vi "run_pharmaBotExp_v0.015.vi"(0 "data in":T12={"daq_ao 1"="Dev1/ao0", "daq_ai 1"="Dev1/ai0", "experiment day folder"=path "C:/multiBot/data/debug/testing", "Multiclamp init error"=0, "Multiclamp Handle Out"=10225184, "sampling rate (Hz)"=20000, "trial name"="t1"}, 1 "auto run?":bool=TRUE, 3 "which manipulator":T13(ring), 4 "HEK/slice options":enum16{"slice", "HEK"}(ring), 5 "error in":errorcluster, 6 "Validate after Experiment":bool, 7 "common cluster":T9, 11 "individual controls in":T8, 13 "images":T3={"slice image"="remote image 000000001461186C", "pipette template"="remote image 000000001461152C", "found pipette"=refnum, "pipette mask for cell tracker"=refnum, "cell images ref"=refnum}) -> (10 "Cell Looks Good?":bool=TRUE, 12 "ValidationOutputCluster":T5(array[cluster]), 14 "ValidationResults":waveform(dbl)[][](array[waveform]), 15 "ValidationPos1":T6(array[ring]), 16 "Exp. Terminated":bool, 17 "ValidationPos2":T6(array[ring]), 18 "ValidationWaveform":waveform(dbl)[](array[waveform]), 19 "error out":errorcluster)   [LabVIEW 2015] (continued)
  T24 = cluster{"Which Position to use for Experiment":enum16{"Jumper Safe Position", "Experiment Safe Position", "Jumper Position A", "Jumper Position B", "Jumper Position C", "Jumper Position o-A", "Jumper Position A-o", "Jumper Position A-B", "Jumper Position B-A", "Jumper Position B-C", "Jumper Position C-B", "Jumper Position C-o", "Jumper Position o-C", "Don't Move"}, "Duration (s)":dbl, "Delay (s)":dbl, "Ramp Slope (mV/s)":dbl, "Voltage Start (mV)":dbl, "Replicates":dbl, "Voltage End (mV)":dbl, "Ramp Duration (s)":dbl, "Vholding (mV)":dbl, "Valve 1 Position":i16, "Valve 2 Position":i16, "Valve 3 Position":i16, "valve 1 used now?":bool, "valve 2 used now?":bool, "valve 3 used now? ":bool, "Maintain Final Voltage until end?":bool, "protocol Preview":waveform(dbl)[]}
  T25 = cluster{"Which Position to use for Experiment":enum16{"Jumper Safe Position", "Experiment Safe Position", "Jumper Position A", "Jumper Position B", "Jumper Position C", "Jumper Position o-A", "Jumper Position A-o", "Jumper Position A-B", "Jumper Position B-A", "Jumper Position B-C", "Jumper Position C-B", "Jumper Position C-o", "Jumper Position o-C", "Don't Move"}, "Duration (s)":dbl, "Delay (s)":dbl, "Pulse 2 (s)":dbl, "Pulse 1 (mV)":dbl, "Replicates":dbl, "Pulse 1 (s)":dbl, "Pulse 2 (mV)":dbl, "Vholding (mV)":dbl, "Valve 1 Position":i16, "Valve 2 Position":i16, "Valve 3 Position":i16, "valve 1 used now?":bool, "valve 2 used now?":bool, "valve 3 used now? ":bool, "Maintain Final Voltage until end?":bool, "delta Pulse 1 (mV)":dbl, "delta Pulse 2 (mV)":dbl, "Sweeps":dbl, "Final Pulse 1 (mV)":dbl, "Final Pulse 2 (mV)":dbl, "protocol Preview":waveform(dbl)[]}
  T26 = cluster{"Which Position to use for Experiment":enum16{"Jumper Safe Position", "Experiment Safe Position", "Jumper Position A", "Jumper Position B", "Jumper Position C", "Jumper Position o-A", "Jumper Position A-o", "Jumper Position A-B", "Jumper Position B-A", "Jumper Position B-C", "Jumper Position C-B", "Jumper Position C-o", "Jumper Position o-C", "Don't Move"}, "Start Position (N)":string, "Jump Position (m)":string, "Duration (s)":dbl, "Delay (s)":dbl, "Pulse Width (s)":dbl, "Valve 1 Position":i16, "Valve 2 Position":i16, "Replicates":dbl, "Pulse Period (s)":dbl, "Vholding (mV)":dbl, "Number of Pulses":dbl, "valve 1 used now?":bool, "valve 2 used now?":bool, "valve 3 used now? ":bool, "Valve 3 Position":i16, "protocol Preview":waveform(dbl)[]}
  T27 = cluster{"Which Position to use for Experiment":enum16{"Jumper Safe Position", "Experiment Safe Position", "Jumper Position A", "Jumper Position B", "Jumper Position C", "Jumper Position o-A", "Jumper Position A-o", "Jumper Position A-B", "Jumper Position B-A", "Jumper Position B-C", "Jumper Position C-B", "Jumper Position C-o", "Jumper Position o-C", "Don't Move"}, "Start Position (N)":string, "Jump Position (m)":string, "Duration (s)":dbl, "Delay (s)":dbl, "Pulse Width (s)":dbl, "Replicates":dbl, "Pulse Delay (s)":dbl, "Pulse Delta Delay (s)":dbl, "Vholding (mV)":dbl, "Valve 1 Position":i16, "Valve 2 Position":i16, "valve 1 used now?":bool, "valve 2 used now?":bool, "valve 3 used now? ":bool, "Valve 3 Position":i16, "protocol Preview":waveform(dbl)[]}
  T28 = cluster{"Start Position (N)":enum16{"Jumper Safe Position", "Experiment Safe Position", "Jumper Position A", "Jumper Position B", "Jumper Position C", "Jumper Position o-A", "Jumper Position A-o", "Jumper Position A-B", "Jumper Position B-A", "Jumper Position B-C", "Jumper Position C-B", "Jumper Position C-o", "Jumper Position o-C", "Don't Move"}, "Duration (s)":dbl, "Delay (s)":dbl, "Pulse Width (s)":dbl, "Valve 1 Position":i16, "Valve 2 Position":i16, "Replicates":dbl, "Jump Position (m)":enum16{"Jumper Safe Position", "Experiment Safe Position", "Jumper Position A", "Jumper Position B", "Jumper Position C", "Jumper Position o-A", "Jumper Position A-o", "Jumper Position A-B", "Jumper Position B-A", "Jumper Position B-C", "Jumper Position C-B", "Jumper Position C-o", "Jumper Position o-C", "Don't Move"}, "Vholding (mV)":dbl, "Valve 3 Position":i16, "valve 1 used now?":bool, "valve 2 used now?":bool, "valve 3 used now? ":bool, "protocol Preview":waveform(dbl)[]}
  T29 = cluster{"Which Position to use for Experiment":enum16{"Jumper Safe Position", "Experiment Safe Position", "Jumper Position A", "Jumper Position B", "Jumper Position C", "Jumper Position o-A", "Jumper Position A-o", "Jumper Position A-B", "Jumper Position B-A", "Jumper Position B-C", "Jumper Position C-B", "Jumper Position C-o", "Jumper Position o-C", "Don't Move"}, "Duration (s)":dbl, "Valve 1 Position":i16, "Valve 2 Position":i16, "Replicates":dbl, "Vholding (mV)":dbl, "Valve 3 Position":i16, "valve 1 used now?":bool, "valve 2 used now?":bool, "valve 3 used now? ":bool, "Record During Solution Change?":bool}
  T30 = cluster{"Start Position (N)":enum16{"Jumper Safe Position", "Experiment Safe Position", "Jumper Position A", "Jumper Position B", "Jumper Position C", "Jumper Position o-A", "Jumper Position A-o", "Jumper Position A-B", "Jumper Position B-A", "Jumper Position B-C", "Jumper Position C-B", "Jumper Position C-o", "Jumper Position o-C"}, "Duration (s)":dbl, "Delay (s)":dbl, "Valve 1 Position":i16, "Valve 2 Position":i16, "Replicates":dbl, "Vholding (mV)":dbl, "Valve 3 Position":i16, "valve 1 used now?":bool, "valve 2 used now?":bool, "valve 3 used now? ":bool, "Jump Position Array":enum16{"Jumper Safe Position", "Experiment Safe Position", "Jumper Position A", "Jumper Position B", "Jumper Position C", "Jumper Position o-A", "Jumper Position A-o", "Jumper Position A-B", "Jumper Position B-A", "Jumper Position B-C", "Jumper Position C-B", "Jumper Position C-o", "Jumper Position o-C"}[], "Position Dwell Time (s)":dbl[], "protocol Preview":waveform(dbl)[]}
  T31 = cluster{"Which Position to use for Experiment":enum16{"Jumper Safe Position", "Experiment Safe Position", "Jumper Position A", "Jumper Position B", "Jumper Position C", "Jumper Position o-A", "Jumper Position A-o", "Jumper Position A-B", "Jumper Position B-A", "Jumper Position B-C", "Jumper Position C-B", "Jumper Position C-o", "Jumper Position o-C", "Don't Move"}, "Duration (s)":dbl, "Delay (s)":dbl, "Pulse 2 (s)":dbl, "Pulse 1 (pA)":dbl, "Replicates":dbl, "Pulse 1 (s)":dbl, "Pulse 2 (pA)":dbl, "Iholding (pA)":dbl, "Valve 1 Position":i16, "Valve 2 Position":i16, "Valve 3 Position":i16, "valve 1 used now?":bool, "valve 2 used now?":bool, "valve 3 used now? ":bool, "Maintain Final Voltage until end?":bool, "delta Pulse 1 (pA)":dbl, "delta Pulse 2 (pA)":dbl, "Sweeps":dbl, "Final Pulse 1 (pA)":dbl, "Final Pulse 2 (pA)":dbl, "protocol Preview":waveform(dbl)[]}
  T32 = cluster{"Which Position to use for Experiment":enum16{"Jumper Safe Position", "Experiment Safe Position", "Jumper Position A", "Jumper Position B", "Jumper Position C", "Jumper Position o-A", "Jumper Position A-o", "Jumper Position A-B", "Jumper Position B-A", "Jumper Position B-C", "Jumper Position C-B", "Jumper Position C-o", "Jumper Position o-C", "Don't Move"}, "Duration (s)":dbl, "Delay (s)":dbl, "Ramp Slope (pA/s)":dbl, "Current Start (pA)":dbl, "Replicates":dbl, "Current End (pA)":dbl, "Ramp Duration (s)":dbl, "Iholding (pA)":dbl, "Valve 1 Position":i16, "Valve 2 Position":i16, "Valve 3 Position":i16, "valve 1 used now?":bool, "valve 2 used now?":bool, "valve 3 used now? ":bool, "Maintain Final Voltage until end?":bool, "protocol Preview":waveform(dbl)[]}
  T33 = cluster{"Which Position to use for Experiment":enum16{"Jumper Safe Position", "Experiment Safe Position", "Jumper Position A", "Jumper Position B", "Jumper Position C", "Jumper Position o-A", "Jumper Position A-o", "Jumper Position A-B", "Jumper Position B-A", "Jumper Position B-C", "Jumper Position C-B", "Jumper Position C-o", "Jumper Position o-C", "Don't Move"}, "Duration (s)":dbl, "Valve 1 Position":i16, "Valve 2 Position":i16, "Replicates":dbl, "Iholding (pA)":dbl, "Valve 3 Position":i16, "valve 1 used now?":bool, "valve 2 used now?":bool, "valve 3 used now? ":bool, "Record During Solution Change?":bool}
  T34 = cluster{"Phase A Done":refnum<vi>, "Phase B Done":refnum<vi>, "Phase C Done":refnum<vi>, "Phase D Done":refnum<vi>, "Phase E Done":refnum<vi>, "Phase F Done":refnum<vi>, "Phase G Done":refnum<vi>, "Phase H Done":refnum<vi>, "Phase I Done":refnum<vi>, "Phase J Done":refnum<vi>, "Phase K Done":refnum<vi>, "Phase L Done":refnum<vi>}
  T35 = cluster{"time of Last V1 Change":refnum<vi>, "time of Last V2 Change":refnum<vi>, "time of Last V3 Change":refnum<vi>}
  T36 = typedef "transform_cluster_actuator.ctl" = cluster{"s":refnum<vi>, "manip 1":refnum<vi>, "manip 2":refnum<vi>, "manip 3":refnum<vi>, "manip 4":refnum<vi>}
  T37 = typedef "transform_properties_actuators.ctl" = cluster{"theta (deg)":dbl, "X sc factor (px/step)":dbl, "Y sc factor (px/step)":dbl, "zero loc (x,y,z)":dbl[], "flip y?":bool, "flip x?":bool, "gamma (deg)":dbl, "flip z?":bool, "Z sc factor (px/step)":dbl, "actuator":T38, "safe space (steps)":i32[]}
  T38 = typedef "actuator_cluster.ctl" = cluster{"Actuator COM":refnum<visa-resource-name>, "Actuator type":T39}
  T39 = typedef "actuator_type.ctl" = enum16{"Scientifica", "Sutter", "Demo", "Off"}
  T40 = typedef "RWC_Actions.ctl" = enum16{"Read", "Write", "Read and Create"}
  T41 = enum16{"open", "replace", "create", "open or create", "replace or create", "replace or create with confirmation"}
  T42 = enum16{"Jumper Safe Position", "Experiment Safe Position", "Jumper Position A", "Jumper Position B", "Jumper Position C", "Jumper Position o-A", "Jumper Position A-o", "Jumper Position A-B", "Jumper Position B-A", "Jumper Position B-C", "Jumper Position C-B", "Jumper Position C-o", "Jumper Position o-C"}
  T43 = typedef "NI_AALBase.lvlib/Filter Passband Type.ctl" = enum32{"Lowpass", "Highpass", "Bandpass", "Bandstop"}
  T44 = enum32{"Invalid", "Standard", "Closed", "Hidden", "Minimized", "Maximized"}
  T45 = typedef "pressure_box_control.ctl" = cluster{"Pressure box COM":refnum<visa-resource-name>, "pressure box type":T46, "High pos pressure (mBar)":dbl, "Low pos pressure (mBar)":dbl, "Vacuum pressure (mBar)":dbl, "calibration":enum16{"PA_vacPump", "PA_venturi", "Neuromatics", "ilyaRig", "mightenRig"}}
  T46 = typedef "pressure_box_type.ctl" = enum16{"Neuromatics", "ProportionAir", "Demo box", "N-ProportionAir"}
diagram:
  w338 = FALSE ("Phase A")
  w339 = "" ("Phase A Exp Option")
  w340 = FALSE ("Phase A")
  # "ValidatePositions & Clean?"
  # "Analyze\nInitial\nData"
  # "SaveConfig"
  # "EndingSet"
  # "RunExperiment"
  # "StartingSet"
  # "Run QC"
  # "Move To Experiment \n          safe space"
  # "Lift Cell"
  # "RUN AUTO WC"
  # "initializing"
  # "Initalization"
  # "HEK/slice options = \"\\14\\00€\\00\\00\\00\\00\\01\\00#@\\16\\00\\02\\05slice\\03HEK\\00\\11HEK/slice options\\00\\01\\00\\00\\00\\01\\00\\00\\00\\00\"\nHEK/slice options string = \"\\14\\00€\\00\\00\\00\\00\\01\\00\"@0ÿÿÿÿ\\18HEK/slice options string\\00\\00\\01\\00\\00\\00\\00\\00\\03HEK\\00\\00\\00\\00\""
  # "PLOTS"
  # "MISC"
  # "create reference for vclamp, iclamp plots\nsave as folder"
  # "load initial values"
  # "HOLDING"
  # "repMemTest"
  n1 = control-ref of="Jump Train G"() -> (w91:refnum<vi>)
  n2 = control-ref of="Paired Pulse G"() -> (w92:refnum<vi>)
  n3 = control-ref of="Voltage Ramp G"() -> (w90:refnum<vi>)
  n4 = control-ref of="Voltage Step G"() -> (w89:refnum<vi>)
  n5 = control-ref of="Solution Change G"() -> (w88:refnum<vi>)
  n6 = control-ref of="Single Jump G"() -> (w87:refnum<vi>)
  n7 = control-ref of="Single Manip Jump G"() -> (w86:refnum<vi>)
  n8 = control-ref of="Current Pulse G"() -> (w22:refnum<vi>)
  n9 = control-ref of="Current Ramp G"() -> (w21:refnum<vi>)
  n10 = control-ref of="Gap Free Iclamp G"() -> (w20:refnum<vi>)
  n11 = control-ref of="Gap Free G"() -> (w85:refnum<vi>)
  n12 = control-ref of="Multi Manip Jump G"() -> (w84:refnum<vi>)
  n13 = control-ref of="Voltage Pulse G"() -> (w83:refnum<vi>)
  n14 = control-ref of="PhaseG Experiment Option"() -> (w352:refnum<vi>)
  n15 = control-ref of="PhaseA Experiment Option"() -> (w390:refnum<vi>)
  n16 = control-ref of="Gap Free Iclamp A"() -> (w38:refnum<vi>)
  n17 = control-ref of="Current Ramp A"() -> (w39:refnum<vi>)
  n18 = control-ref of="Current Pulse A"() -> (w40:refnum<vi>)
  n19 = control-ref of="Multi Manip Jump A"() -> (w311:refnum<vi>)
  n20 = control-ref of="Single Manip Jump A"() -> (w309:refnum<vi>)
  n21 = control-ref of="Voltage Pulse A"() -> (w312:refnum<vi>)
  n22 = control-ref of="Gap Free A"() -> (w310:refnum<vi>)
  n23 = control-ref of="Paired Pulse A"() -> (w303:refnum<vi>)
  n24 = control-ref of="Voltage Ramp A"() -> (w305:refnum<vi>)
  n25 = control-ref of="Voltage Step A"() -> (w306:refnum<vi>)
  n26 = control-ref of="Solution Change A"() -> (w307:refnum<vi>)
  n27 = control-ref of="Single Jump A"() -> (w308:refnum<vi>)
  n28 = control-ref of="Jump Train A"() -> (w304:refnum<vi>)
  n29 = control-ref of="Jump Train H"() -> (w101:refnum<vi>)
  n30 = control-ref of="Paired Pulse H"() -> (w102:refnum<vi>)
  n31 = control-ref of="Voltage Ramp H"() -> (w100:refnum<vi>)
  n32 = control-ref of="Voltage Step H"() -> (w99:refnum<vi>)
  n33 = control-ref of="Solution Change H"() -> (w98:refnum<vi>)
  n34 = control-ref of="Single Jump H"() -> (w97:refnum<vi>)
  n35 = control-ref of="Single Manip Jump H"() -> (w96:refnum<vi>)
  n36 = control-ref of="Gap Free H"() -> (w95:refnum<vi>)
  n37 = control-ref of="Multi Manip Jump H"() -> (w94:refnum<vi>)
  n38 = control-ref of="Voltage Pulse H"() -> (w93:refnum<vi>)
  n39 = control-ref of="Current Pulse H"() -> (w19:refnum<vi>)
  n40 = control-ref of="Current Ramp H"() -> (w18:refnum<vi>)
  n41 = control-ref of="Gap Free Iclamp H"() -> (w17:refnum<vi>)
  n42 = Build Array(w352, w92, w91, w90, w89, w88, w87, w86, w85, w84, w83, w22, w21, w20) -> (w346:refnum<vi>[])
  n43 = control-ref of="PhaseH Experiment Option"() -> (w351:refnum<vi>)
  n44 = control-ref of="PhaseB Experiment Option"() -> (w389:refnum<vi>)
  n45 = Build Array(w390, w303, w304, w305, w306, w307, w308, w309, w310, w311, w312, w40, w39, w38) -> (w384:refnum<vi>[])
  n46 = control-ref of="Paired Pulse B"() -> (w292:refnum<vi>)
  n47 = control-ref of="Jump Train B"() -> (w291:refnum<vi>)
  n48 = control-ref of="Voltage Ramp B"() -> (w290:refnum<vi>)
  n49 = control-ref of="Voltage Step B"() -> (w289:refnum<vi>)
  n50 = control-ref of="Solution Change B"() -> (w288:refnum<vi>)
  n51 = control-ref of="Single Jump B"() -> (w287:refnum<vi>)
  n52 = control-ref of="Single Manip Jump B"() -> (w286:refnum<vi>)
  n53 = control-ref of="Gap Free B"() -> (w285:refnum<vi>)
  n54 = control-ref of="Multi Manip Jump B"() -> (w284:refnum<vi>)
  n55 = control-ref of="Voltage Pulse B"() -> (w283:refnum<vi>)
  n56 = control-ref of="Current Pulse B"() -> (w37:refnum<vi>)
  n57 = control-ref of="Current Ramp B"() -> (w36:refnum<vi>)
  n58 = control-ref of="Gap Free Iclamp B"() -> (w35:refnum<vi>)
  n59 = control-ref of="A Solution1"() -> (w419:refnum<vi>)
  n60 = control-ref of="A Solution2"() -> (w418:refnum<vi>)
  n61 = control-ref of="A Solution3"() -> (w417:refnum<vi>)
  n62 = control-ref of="A Solution4"() -> (w416:refnum<vi>)
  n63 = control-ref of="A Solution5"() -> (w415:refnum<vi>)
  n64 = control-ref of="A Solution6"() -> (w414:refnum<vi>)
  n65 = control-ref of="A Solution7"() -> (w413:refnum<vi>)
  n66 = control-ref of="A Solution8"() -> (w412:refnum<vi>)
  n67 = control-ref of="Jump Train I"() -> (w111:refnum<vi>)
  n68 = control-ref of="Paired Pulse I"() -> (w112:refnum<vi>)
  n69 = control-ref of="Voltage Ramp I"() -> (w110:refnum<vi>)
  n70 = control-ref of="Voltage Step I"() -> (w109:refnum<vi>)
  n71 = control-ref of="Solution Change I"() -> (w108:refnum<vi>)
  n72 = control-ref of="Single Jump I"() -> (w107:refnum<vi>)
  n73 = control-ref of="Single Manip Jump I"() -> (w106:refnum<vi>)
  n74 = control-ref of="Gap Free I"() -> (w105:refnum<vi>)
  n75 = control-ref of="Multi Manip Jump I"() -> (w104:refnum<vi>)
  n76 = control-ref of="Voltage Pulse I"() -> (w103:refnum<vi>)
  n77 = control-ref of="Current Pulse I"() -> (w16:refnum<vi>)
  n78 = control-ref of="Current Ramp I"() -> (w15:refnum<vi>)
  n79 = control-ref of="Gap Free Iclamp I"() -> (w14:refnum<vi>)
  n80 = control-ref of="PhaseI Experiment Option"() -> (w350:refnum<vi>)
  n81 = Build Array(w351, w102, w101, w100, w99, w98, w97, w96, w95, w94, w93, w19, w18, w17) -> (w345:refnum<vi>[])
  n82 = control-ref of="Paired Pulse C"() -> (w272:refnum<vi>)
  n83 = control-ref of="Jump Train C"() -> (w271:refnum<vi>)
  n84 = control-ref of="Voltage Ramp C"() -> (w270:refnum<vi>)
  n85 = control-ref of="Voltage Step C"() -> (w269:refnum<vi>)
  n86 = control-ref of="Solution Change C"() -> (w268:refnum<vi>)
  n87 = control-ref of="Single Jump C"() -> (w267:refnum<vi>)
  n88 = control-ref of="Single Manip Jump C"() -> (w266:refnum<vi>)
  n89 = control-ref of="Gap Free C"() -> (w265:refnum<vi>)
  n90 = control-ref of="Multi Manip Jump C"() -> (w264:refnum<vi>)
  n91 = control-ref of="Current Pulse C"() -> (w34:refnum<vi>)
  n92 = control-ref of="Current Ramp C"() -> (w33:refnum<vi>)
  n93 = control-ref of="Gap Free Iclamp C"() -> (w32:refnum<vi>)
  n94 = control-ref of="Voltage Pulse C"() -> (w263:refnum<vi>)
  n95 = control-ref of="PhaseC Experiment Option"() -> (w388:refnum<vi>)
  n96 = Build Array(w389, w292, w291, w290, w289, w288, w287, w286, w285, w284, w283, w37, w36, w35) -> (w383:refnum<vi>[])
  n97 = Build Array(w419, w418, w417, w416, w415, w414, w413, w412) -> (w411:refnum<vi>[])
  n98 = control-ref of="Paired Pulse J"() -> (w122:refnum<vi>)
  n99 = control-ref of="Single Manip Jump J"() -> (w116:refnum<vi>)
  n100 = control-ref of="Voltage Ramp J"() -> (w120:refnum<vi>)
  n101 = control-ref of="Voltage Step J"() -> (w119:refnum<vi>)
  n102 = control-ref of="Solution Change J"() -> (w118:refnum<vi>)
  n103 = control-ref of="Single Jump J"() -> (w117:refnum<vi>)
  n104 = control-ref of="Jump Train J"() -> (w121:refnum<vi>)
  n105 = control-ref of="Gap Free J"() -> (w115:refnum<vi>)
  n106 = control-ref of="Multi Manip Jump J"() -> (w114:refnum<vi>)
  n107 = control-ref of="Voltage Pulse J"() -> (w113:refnum<vi>)
  n108 = control-ref of="Current Pulse J"() -> (w13:refnum<vi>)
  n109 = control-ref of="Current Ramp J"() -> (w12:refnum<vi>)
  n110 = control-ref of="Gap Free Iclamp J"() -> (w11:refnum<vi>)
  n111 = control-ref of="B Solution1"() -> (w409:refnum<vi>)
  n112 = control-ref of="B Solution2"() -> (w405:refnum<vi>)
  n113 = control-ref of="B Solution3"() -> (w404:refnum<vi>)
  n114 = control-ref of="B Solution4"() -> (w403:refnum<vi>)
  n115 = control-ref of="B Solution5"() -> (w402:refnum<vi>)
  n116 = control-ref of="B Solution6"() -> (w406:refnum<vi>)
  n117 = control-ref of="B Solution7"() -> (w407:refnum<vi>)
  n118 = control-ref of="B Solution8"() -> (w408:refnum<vi>)
  n119 = Build Array(w350, w112, w111, w110, w109, w108, w107, w106, w105, w104, w103, w16, w15, w14) -> (w344:refnum<vi>[])
  n120 = control-ref of="PhaseD Experiment Option"() -> (w387:refnum<vi>)
  n121 = control-ref of="PhaseJ Experiment Option"() -> (w349:refnum<vi>)
  n122 = Build Array(w388, w272, w271, w270, w269, w268, w267, w266, w265, w264, w263, w34, w33, w32) -> (w382:refnum<vi>[])
  n123 = control-ref of="Current Pulse D"() -> (w31:refnum<vi>)
  n124 = control-ref of="Current Ramp D"() -> (w30:refnum<vi>)
  n125 = control-ref of="Gap Free Iclamp D"() -> (w29:refnum<vi>)
  n126 = control-ref of="Paired Pulse D"() -> (w252:refnum<vi>)
  n127 = control-ref of="Jump Train D"() -> (w251:refnum<vi>)
  n128 = control-ref of="Voltage Ramp D"() -> (w250:refnum<vi>)
  n129 = control-ref of="Voltage Step D"() -> (w249:refnum<vi>)
  n130 = control-ref of="Solution Change D"() -> (w248:refnum<vi>)
  n131 = control-ref of="Single Jump D"() -> (w247:refnum<vi>)
  n132 = control-ref of="Single Manip Jump D"() -> (w246:refnum<vi>)
  n133 = control-ref of="Gap Free D"() -> (w245:refnum<vi>)
  n134 = control-ref of="Multi Manip Jump D"() -> (w244:refnum<vi>)
  n135 = control-ref of="Voltage Pulse D"() -> (w243:refnum<vi>)
  n136 = Build Array(w409, w405, w404, w403, w402, w406, w407, w408) -> (w401:refnum<vi>[])
  n137 = control-ref of="PhaseE Experiment Option"() -> (w386:refnum<vi>)
  n138 = Build Array(w387, w252, w251, w250, w249, w248, w247, w246, w245, w244, w243, w31, w30, w29) -> (w381:refnum<vi>[])
  n139 = Build Array(w349, w122, w121, w120, w119, w118, w117, w116, w115, w114, w113, w13, w12, w11) -> (w343:refnum<vi>[])
  n140 = control-ref of="PhaseK Experiment Option"() -> (w348:refnum<vi>)
  n141 = control-ref of="Paired Pulse K"() -> (w123:refnum<vi>)
  n142 = control-ref of="Single Manip Jump K"() -> (w129:refnum<vi>)
  n143 = control-ref of="Voltage Ramp K"() -> (w125:refnum<vi>)
  n144 = control-ref of="Voltage Step K"() -> (w126:refnum<vi>)
  n145 = control-ref of="Solution Change K"() -> (w127:refnum<vi>)
  n146 = control-ref of="Single Jump K"() -> (w128:refnum<vi>)
  n147 = control-ref of="Jump Train K"() -> (w124:refnum<vi>)
  n148 = control-ref of="Gap Free K"() -> (w130:refnum<vi>)
  n149 = control-ref of="Multi Manip Jump K"() -> (w131:refnum<vi>)
  n150 = control-ref of="Voltage Pulse K"() -> (w132:refnum<vi>)
  n151 = control-ref of="Current Pulse E"() -> (w28:refnum<vi>)
  n152 = control-ref of="Current Ramp E"() -> (w27:refnum<vi>)
  n153 = control-ref of="Gap Free Iclamp E"() -> (w26:refnum<vi>)
  n154 = control-ref of="Current Pulse K"() -> (w10:refnum<vi>)
  n155 = control-ref of="Current Ramp K"() -> (w9:refnum<vi>)
  n156 = control-ref of="Gap Free Iclamp K"() -> (w8:refnum<vi>)
  n157 = control-ref of="Jump Train E"() -> (w231:refnum<vi>)
  n158 = control-ref of="Voltage Ramp E"() -> (w230:refnum<vi>)
  n159 = control-ref of="Voltage Step E"() -> (w229:refnum<vi>)
  n160 = control-ref of="Solution Change E"() -> (w228:refnum<vi>)
  n161 = control-ref of="Single Jump E"() -> (w227:refnum<vi>)
  n162 = control-ref of="Single Manip Jump E"() -> (w226:refnum<vi>)
  n163 = control-ref of="Gap Free E"() -> (w225:refnum<vi>)
  n164 = control-ref of="Multi Manip Jump E"() -> (w224:refnum<vi>)
  n165 = control-ref of="Voltage Pulse E"() -> (w223:refnum<vi>)
  n166 = control-ref of="Paired Pulse E"() -> (w232:refnum<vi>)
  n167 = control-ref of="C Solution1"() -> (w399:refnum<vi>)
  n168 = control-ref of="C Solution2"() -> (w398:refnum<vi>)
  n169 = control-ref of="C Solution3"() -> (w397:refnum<vi>)
  n170 = control-ref of="C Solution4"() -> (w396:refnum<vi>)
  n171 = control-ref of="C Solution5"() -> (w395:refnum<vi>)
  n172 = control-ref of="C Solution6"() -> (w394:refnum<vi>)
  n173 = control-ref of="C Solution7"() -> (w393:refnum<vi>)
  n174 = control-ref of="C Solution8"() -> (w392:refnum<vi>)
  n175 = control-ref of="Command steps (mV)"() -> (w459:refnum<vi>)
  n176 = control-ref of="Command steps (pA)"() -> (w464:refnum<vi>)
  n177 = control-ref of="Recorded currents (pA)"() -> (w463:refnum<vi>)
  n178 = control-ref of="Recorded voltage (mV)"() -> (w462:refnum<vi>)
  n179 = Build Array(w399, w398, w397, w396, w395, w394, w393, w392) -> (w391:refnum<vi>[])
  n180 = Build Array(w348, w123, w124, w125, w126, w127, w128, w129, w130, w131, w132, w10, w9, w8) -> (w342:refnum<vi>[])
  n181 = control-ref of="PhaseF Experiment Option"() -> (w385:refnum<vi>)
  n182 = Build Array(w386, w232, w231, w230, w229, w228, w227, w226, w225, w224, w223, w28, w27, w26) -> (w380:refnum<vi>[])
  n183 = control-ref of="holding memtest"() -> (w467:refnum<vi>)
  n184 = control-ref of="Paired Pulse L"() -> (w142:refnum<vi>)
  n185 = control-ref of="Single Manip Jump L"() -> (w136:refnum<vi>)
  n186 = control-ref of="Current Pulse F"() -> (w25:refnum<vi>)
  n187 = control-ref of="Current Ramp F"() -> (w24:refnum<vi>)
  n188 = control-ref of="Gap Free Iclamp F"() -> (w23:refnum<vi>)
  n189 = control-ref of="Voltage Ramp L"() -> (w140:refnum<vi>)
  n190 = control-ref of="Voltage Step L"() -> (w139:refnum<vi>)
  n191 = control-ref of="Solution Change L"() -> (w138:refnum<vi>)
  n192 = control-ref of="Single Jump L"() -> (w137:refnum<vi>)
  n193 = control-ref of="Jump Train L"() -> (w141:refnum<vi>)
  n194 = control-ref of="Paired Pulse F"() -> (w152:refnum<vi>)
  n195 = control-ref of="Jump Train F"() -> (w151:refnum<vi>)
  n196 = control-ref of="Voltage Ramp F"() -> (w150:refnum<vi>)
  n197 = control-ref of="Voltage Step F"() -> (w149:refnum<vi>)
  n198 = control-ref of="Solution Change F"() -> (w148:refnum<vi>)
  n199 = control-ref of="Single Jump F"() -> (w147:refnum<vi>)
  n200 = control-ref of="Single Manip Jump F"() -> (w146:refnum<vi>)
  n201 = control-ref of="Gap Free F"() -> (w145:refnum<vi>)
  n202 = control-ref of="Multi Manip Jump F"() -> (w144:refnum<vi>)
  n203 = control-ref of="Voltage Pulse F"() -> (w143:refnum<vi>)
  n204 = control-ref of="repMemTest Iprot"() -> (w486:refnum<vi>)
  n205 = control-ref of="repMemTest Vprot"() -> (w485:refnum<vi>)
  n206 = control-ref of="repMemTest Iclamp memtest"() -> (w484:refnum<vi>)
  n207 = control-ref of="repMemTest Vclamp memtest"() -> (w483:refnum<vi>)
  n208 = control-ref of="repMemTest sets"() -> (w487:refnum<vi>)
  n209 = control-ref of="holding Iclamp memtest"() -> (w469:refnum<vi>)
  n210 = control-ref of="holding Vclamp memtest"() -> (w468:refnum<vi>)
  n211 = control-ref of="cell stats"() -> (w465:refnum<vi>)
  n212 = control-ref of="Gap Free L"() -> (w135:refnum<vi>)
  n213 = control-ref of="wait after init (s)"() -> (w488:refnum<vi>)
  n214 = control-ref of="wait after repMemTest set (s)"() -> (w489:refnum<vi>)
  n215 = control-ref of="Multi Manip Jump L"() -> (w134:refnum<vi>)
  n216 = control-ref of="Voltage Pulse L"() -> (w133:refnum<vi>)
  n217 = control-ref of="Current Pulse L"() -> (w7:refnum<vi>)
  n218 = control-ref of="Current Ramp L"() -> (w6:refnum<vi>)
  n219 = control-ref of="Gap Free Iclamp L"() -> (w5:refnum<vi>)
  n220 = control-ref of="status"() -> (w466:refnum<vi>)
  n221 = control-ref of="trial comments"() -> (w461:refnum<vi>)
  n222 = control-ref of="release notes"() -> (w460:refnum<vi>)
  n223 = control-ref of="PhaseL Experiment Option"() -> (w347:refnum<vi>)
  n224 = control-ref of="config file"() -> ()  [unwired: 1 out]
  n225 = control-ref of="Validate after Experiment"() -> (w2:refnum<vi>)
  n226 = control-ref of="twitter?"() -> (w4:refnum<vi>)
  n227 = control-ref of="Don't Lift?"() -> (w3:refnum<vi>)
  n228 = control-ref of="Lane C Controlled by which valve?"() -> (w400:refnum<vi>)
  n229 = control-ref of="Lane A Controlled by which valve?"() -> (w420:refnum<vi>)
  n230 = control-ref of="Lane B Controlled by which valve?"() -> (w410:refnum<vi>)
  n231 = control-ref of="How Many Experimental Phases?"() -> (w422:refnum<vi>)
  n232 = control-ref of="Lift Cell (T, F-Pull Patch)?"() -> (w421:refnum<vi>)
  n233 = Build Array(w385, w152, w151, w150, w149, w148, w147, w146, w145, w144, w143, w25, w24, w23) -> (w379:refnum<vi>[])
  n234 = Build Array(w347, w142, w141, w140, w139, w138, w137, w136, w135, w134, w133, w7, w6, w5) -> (w341:refnum<vi>[])
  n235 = control-ref of="Waveform Simulation sampling rate (Hz)"() -> (w79:refnum<vi>)
  n236 = control-ref of="Waveform Simulation Jump Filter (Hz)"() -> (w77:refnum<vi>)
  n237 = flat-sequence {
    tunnel: "error in" -> [w491]
    tunnel: [w491] -> w80
    tunnel: [TRUE] -> w443
    tunnel: [w496] -> w81
    tunnel: w80 -> [w496]
    frame #0 {
      w492 = FALSE ("Running")
      w490 = FALSE ("Running")
      w494 = FALSE ("Experiment Done")
      n238 = local write "Terminate Experiment"(w490) -> ()
      n239 = property on="Experiment Done" class="Bool (strict)"("Value"=w494) -> ()  [unwired: 2 in, 2 out]
      n240 = property on="auto WC run trigger" class="Bool (strict)"("Value"=w494) -> ()  [unwired: 2 in, 2 out]
      n241 = property on="status" class="Str"("Value"="") -> ()  [unwired: 2 in, 2 out]
      n242 = local write "run"(w490) -> ()
      n243 = local write "update plots"(w490) -> ()
      n244 = local write "Puase for Loading"(w490) -> ()
      n245 = local write "load"(w490) -> ()
      n246 = local write "Exp. Terminated"(w490) -> ()
      n247 = local write "Running"(w492) -> ()
      n248 = local write "Exp Started"(w492) -> ()
      n249 = Wait (ms)(milliseconds to wait=u32 50) -> ()  [unwired: 1 out]
    }
    frame #1 {
      n250 = Wait (ms)(milliseconds to wait=u32 50) -> ()  [unwired: 1 out]
    }
  }
  n251 = Build Array (concatenate)(w486, w485, w484, w483, w487, w488, w489, w469, w468, w467, w466, w465, w459, w464, w463, w462, w461, w460, w2, w3, w4, w422, w421, w420, w411, w410, w401, w400, w391, w384, w383, w382, w381, w380, w379, w346, w345, w344, w343, w342, w341, w79, w77) -> (w475:refnum<vi>[])
  n252 = call "condition_control_array_v02.vi"("control array in"=w475) -> ("control array out"=w474:refnum<vi>[])  [unwired: 9 in, 1 out]
  n253 = case shown="True" w443 {
    tunnel: w81 -> [w499 w501]
    tunnel: [w499 w500] -> _
    frame False {
    }
    frame True {
      n254 = case shown="True" "auto run?" {
        tunnel: w501 -> [w503 w504]
        tunnel: [w503 w504] -> w500
        frame False {
        }
        frame True {
          n255 = flat-sequence {
            tunnel: [w507] -> w505
            frame #0 {
              n256 = Wait (ms)(milliseconds to wait=u32 1000) -> ()  [unwired: 1 out]
            }
            frame #1 {
              w507 = TRUE ("update plots")
              n257 = local write "Cell Looks Good?"(TRUE ("Cell Looks Good?")) -> ()
              n258 = property on="run" class="Bool (strict)"("Val(Sgnl)"=w507) -> ()  [unwired: 2 in, 2 out]
              n259 = property on="update plots" class="Bool (strict)"("Val(Sgnl)"=w507) -> ()  [unwired: 2 in, 2 out]
            }
          }
          n260 = local write "auto WC run trigger"(w505) -> ()
        }
      }
    }
  }
  n261 = Unbundle By Name("data in") -> ("Multiclamp Handle Out"=w479:u32, "Multiclamp init error"=w478:i32)
  n262 = Unbundle By Name("common cluster") -> ("misc common.stop memtest"=w441:refnum<vi>, "positioning+hunting common.pressure box"=w377:refnum<vi>)
  n263 = Unbundle By Name("data in") -> ("sampling rate (Hz)"=w378:i32)
  n264 = case shown="True" "DEBUG?" {
    tunnel: [w511 w517] -> w481
    tunnel: [w510 w516] -> w480
    tunnel: w479 -> [w511 _]
    tunnel: w478 -> [w510 _]
    tunnel: "data in" -> [w509 w515]
    tunnel: [w509 w514] -> w476
    tunnel: w4 -> [_ w513]
    frame False {
    }
    frame True {
      n265 = call "init multiclamp.vi"() -> ("Error out"=w516:i32, "Multiclamp Handle Out"=w517:u32)  [unwired: 9 in, 1 out]
      n266 = Bundle By Name(cluster=w515, "Multiclamp Handle Out"=w517, "Multiclamp init error"=w516) -> (w514:T12)
      n267 = property class="Bool (strict)"(reference=w513, "Value"=FALSE) -> ()  [unwired: 1 in, 2 out]
    }
  }
  n268 = call "Get Strings from Enum__ogtk.vi"("Enum"="HEK/slice options") -> ("String Value"=→"HEK/slice options string":string)  [unwired: 7 in, 3 out]
  n269 = property on="data in" class="Clust (strict)"("Value"=w476) -> ()  [unwired: 2 in, 2 out]
  n270 = control-ref of="Experiment Selection A"() -> (w457:refnum<vi>)
  n271 = control-ref of="Experiment Selection B"() -> (w454:refnum<vi>)
  n272 = control-ref of="Experiment Selection C"() -> (w448:refnum<vi>)
  n273 = control-ref of="Experiment Selection D"() -> (w431:refnum<vi>)
  n274 = control-ref of="Experiment Selection E"() -> (w430:refnum<vi>)
  n275 = control-ref of="Experiment Selection F"() -> (w429:refnum<vi>)
  n276 = property class="TabCtl (strict)"(reference=w430, "Tabs Visible?"=FALSE) -> ()  [unwired: 1 in, 2 out]
  n277 = property class="TabCtl (strict)"(reference=w429, "Tabs Visible?"=FALSE) -> ()  [unwired: 1 in, 2 out]
  n278 = property class="TabCtl (strict)"(reference=w431, "Tabs Visible?"=FALSE) -> ()  [unwired: 1 in, 2 out]
  n279 = property class="TabCtl (strict)"(reference=w448, "Tabs Visible?"=FALSE) -> ()  [unwired: 1 in, 2 out]
  n280 = property class="TabCtl (strict)"(reference=w457, "Tabs Visible?"=FALSE) -> ()  [unwired: 1 in, 2 out]
  n281 = property class="TabCtl (strict)"(reference=w454, "Tabs Visible?"=FALSE) -> ()  [unwired: 1 in, 2 out]
  n282 = control-ref of="Experiment Selection G"() -> (w365:refnum<vi>)
  n283 = control-ref of="Experiment Selection H"() -> (w368:refnum<vi>)
  n284 = control-ref of="Experiment Selection I"() -> (w369:refnum<vi>)
  n285 = control-ref of="Experiment Selection J"() -> (w374:refnum<vi>)
  n286 = control-ref of="Experiment Selection K"() -> (w375:refnum<vi>)
  n287 = control-ref of="Experiment Selection L"() -> (w376:refnum<vi>)
  n288 = property class="TabCtl (strict)"(reference=w375, "Tabs Visible?"=FALSE) -> ()  [unwired: 1 in, 2 out]
  n289 = property class="TabCtl (strict)"(reference=w376, "Tabs Visible?"=FALSE) -> ()  [unwired: 1 in, 2 out]
  n290 = property class="TabCtl (strict)"(reference=w374, "Tabs Visible?"=FALSE) -> ()  [unwired: 1 in, 2 out]
  n291 = property class="TabCtl (strict)"(reference=w369, "Tabs Visible?"=FALSE) -> ()  [unwired: 1 in, 2 out]
  n292 = property class="TabCtl (strict)"(reference=w365, "Tabs Visible?"=FALSE) -> ()  [unwired: 1 in, 2 out]
  n293 = property class="TabCtl (strict)"(reference=w368, "Tabs Visible?"=FALSE) -> ()  [unwired: 1 in, 2 out]
  n294 = control-ref of="Jump Train G"() -> (w211:refnum<vi>)
  n295 = control-ref of="Paired Pulse G"() -> (w212:refnum<vi>)
  n296 = control-ref of="Voltage Ramp G"() -> (w210:refnum<vi>)
  n297 = control-ref of="Voltage Step G"() -> (w209:refnum<vi>)
  n298 = control-ref of="Solution Change G"() -> (w208:refnum<vi>)
  n299 = control-ref of="Single Jump G"() -> (w207:refnum<vi>)
  n300 = control-ref of="Single Manip Jump G"() -> (w206:refnum<vi>)
  n301 = control-ref of="Multi Manip Jump A"() -> (w314:refnum<vi>)
  n302 = control-ref of="Gap Free Iclamp A"() -> (w74:refnum<vi>)
  n303 = control-ref of="Single Manip Jump A"() -> (w316:refnum<vi>)
  n304 = control-ref of="Gap Free A"() -> (w315:refnum<vi>)
  n305 = control-ref of="Voltage Pulse A"() -> (w313:refnum<vi>)
  n306 = control-ref of="Current Ramp A"() -> (w76:refnum<vi>)
  n307 = control-ref of="Gap Free G"() -> (w205:refnum<vi>)
  n308 = control-ref of="Multi Manip Jump G"() -> (w204:refnum<vi>)
  n309 = control-ref of="Paired Pulse A"() -> (w322:refnum<vi>)
  n310 = control-ref of="Voltage Ramp A"() -> (w320:refnum<vi>)
  n311 = control-ref of="Voltage Step A"() -> (w319:refnum<vi>)
  n312 = control-ref of="Solution Change A"() -> (w318:refnum<vi>)
  n313 = control-ref of="Single Jump A"() -> (w317:refnum<vi>)
  n314 = control-ref of="Current Pulse A"() -> (w75:refnum<vi>)
  n315 = control-ref of="Voltage Pulse G"() -> (w203:refnum<vi>)
  n316 = control-ref of="Jump Train A"() -> (w321:refnum<vi>)
  n317 = control-ref of="Current Pulse G"() -> (w73:refnum<vi>)
  n318 = control-ref of="Current Ramp G"() -> (w72:refnum<vi>)
  n319 = control-ref of="Gap Free Iclamp G"() -> (w71:refnum<vi>)
  n320 = control-ref of="PhaseA Experiment Option"() -> (w453:refnum<vi>)
  n321 = control-ref of="PhaseG Experiment Option"() -> (w364:refnum<vi>)
  n322 = Bundle(cluster="PhaseX Cluster", "Phase Experiment Option"=w364, "Paired Pulse"=w212, "Jump Train"=w211, "Voltage Ramp"=w210, "Voltage Step"=w209, "Solution Change"=w208, "Single Jump"=w207, "Single Manip Jump"=w206, "Gap Free"=w205, "Multi Manip Jump"=w204, "Voltage Pulse"=w203, "Current Pulse"=w73, "Current Ramp"=w72, "Gap Free Iclamp"=w71) -> (w358:T1)
  n323 = Bundle(cluster="PhaseX Cluster", "Phase Experiment Option"=w453, "Paired Pulse"=w322, "Jump Train"=w321, "Voltage Ramp"=w320, "Voltage Step"=w319, "Solution Change"=w318, "Single Jump"=w317, "Single Manip Jump"=w316, "Gap Free"=w315, "Multi Manip Jump"=w314, "Voltage Pulse"=w313, "Current Pulse"=w75, "Current Ramp"=w76, "Gap Free Iclamp"=w74) -> (w450:T1)
  n324 = control-ref of="Jump Train H"() -> (w201:refnum<vi>)
  n325 = control-ref of="Paired Pulse H"() -> (w202:refnum<vi>)
  n326 = control-ref of="Voltage Ramp H"() -> (w200:refnum<vi>)
  n327 = control-ref of="Voltage Step H"() -> (w199:refnum<vi>)
  n328 = control-ref of="Solution Change H"() -> (w198:refnum<vi>)
  n329 = control-ref of="Single Jump H"() -> (w197:refnum<vi>)
  n330 = control-ref of="Single Manip Jump H"() -> (w196:refnum<vi>)
  n331 = control-ref of="Gap Free H"() -> (w195:refnum<vi>)
  n332 = control-ref of="Multi Manip Jump H"() -> (w194:refnum<vi>)
  n333 = control-ref of="Voltage Pulse H"() -> (w193:refnum<vi>)
  n334 = control-ref of="Current Pulse H"() -> (w70:refnum<vi>)
  n335 = control-ref of="Current Ramp H"() -> (w69:refnum<vi>)
  n336 = control-ref of="Gap Free Iclamp H"() -> (w68:refnum<vi>)
  n337 = control-ref of="Current Pulse B"() -> (w67:refnum<vi>)
  n338 = control-ref of="Current Ramp B"() -> (w66:refnum<vi>)
  n339 = control-ref of="Gap Free Iclamp B"() -> (w65:refnum<vi>)
  n340 = control-ref of="Paired Pulse B"() -> (w293:refnum<vi>)
  n341 = control-ref of="Jump Train B"() -> (w294:refnum<vi>)
  n342 = control-ref of="Voltage Ramp B"() -> (w295:refnum<vi>)
  n343 = control-ref of="Voltage Step B"() -> (w296:refnum<vi>)
  n344 = control-ref of="Solution Change B"() -> (w297:refnum<vi>)
  n345 = control-ref of="Single Jump B"() -> (w298:refnum<vi>)
  n346 = control-ref of="Single Manip Jump B"() -> (w299:refnum<vi>)
  n347 = control-ref of="Gap Free B"() -> (w300:refnum<vi>)
  n348 = control-ref of="Multi Manip Jump B"() -> (w301:refnum<vi>)
  n349 = control-ref of="Voltage Pulse B"() -> (w302:refnum<vi>)
  n350 = control-ref of="PhaseB Experiment Option"() -> (w452:refnum<vi>)
  n351 = control-ref of="PhaseH Experiment Option"() -> (w363:refnum<vi>)
  n352 = Bundle(cluster="PhaseX Cluster", "Phase Experiment Option"=w363, "Paired Pulse"=w202, "Jump Train"=w201, "Voltage Ramp"=w200, "Voltage Step"=w199, "Solution Change"=w198, "Single Jump"=w197, "Single Manip Jump"=w196, "Gap Free"=w195, "Multi Manip Jump"=w194, "Voltage Pulse"=w193, "Current Pulse"=w70, "Current Ramp"=w69, "Gap Free Iclamp"=w68) -> (w357:T1)
  n353 = Bundle(cluster="PhaseX Cluster", "Phase Experiment Option"=w452, "Paired Pulse"=w293, "Jump Train"=w294, "Voltage Ramp"=w295, "Voltage Step"=w296, "Solution Change"=w297, "Single Jump"=w298, "Single Manip Jump"=w299, "Gap Free"=w300, "Multi Manip Jump"=w301, "Voltage Pulse"=w302, "Current Pulse"=w67, "Current Ramp"=w66, "Gap Free Iclamp"=w65) -> (w449:T1)
  n354 = control-ref of="Jump Train I"() -> (w191:refnum<vi>)
  n355 = control-ref of="Paired Pulse I"() -> (w192:refnum<vi>)
  n356 = control-ref of="Voltage Ramp I"() -> (w190:refnum<vi>)
  n357 = control-ref of="Voltage Step I"() -> (w189:refnum<vi>)
  n358 = control-ref of="Solution Change I"() -> (w188:refnum<vi>)
  n359 = control-ref of="Single Jump I"() -> (w187:refnum<vi>)
  n360 = control-ref of="Single Manip Jump I"() -> (w186:refnum<vi>)
  n361 = control-ref of="Gap Free I"() -> (w185:refnum<vi>)
  n362 = control-ref of="Multi Manip Jump I"() -> (w184:refnum<vi>)
  n363 = control-ref of="Voltage Pulse I"() -> (w183:refnum<vi>)
  n364 = control-ref of="Current Pulse I"() -> (w58:refnum<vi>)
  n365 = control-ref of="Current Ramp I"() -> (w57:refnum<vi>)
  n366 = control-ref of="Gap Free Iclamp I"() -> (w56:refnum<vi>)
  n367 = control-ref of="PhaseI Experiment Option"() -> (w362:refnum<vi>)
  n368 = control-ref of="PhaseC Experiment Option"() -> (w446:refnum<vi>)
  n369 = control-ref of="Paired Pulse C"() -> (w282:refnum<vi>)
  n370 = control-ref of="Jump Train C"() -> (w281:refnum<vi>)
  n371 = control-ref of="Voltage Ramp C"() -> (w280:refnum<vi>)
  n372 = control-ref of="Voltage Step C"() -> (w279:refnum<vi>)
  n373 = control-ref of="Solution Change C"() -> (w278:refnum<vi>)
  n374 = control-ref of="Single Jump C"() -> (w277:refnum<vi>)
  n375 = control-ref of="Single Manip Jump C"() -> (w276:refnum<vi>)
  n376 = control-ref of="Current Pulse C"() -> (w64:refnum<vi>)
  n377 = control-ref of="Current Ramp C"() -> (w63:refnum<vi>)
  n378 = control-ref of="Gap Free Iclamp C"() -> (w62:refnum<vi>)
  n379 = control-ref of="Gap Free C"() -> (w275:refnum<vi>)
  n380 = control-ref of="Multi Manip Jump C"() -> (w274:refnum<vi>)
  n381 = control-ref of="Voltage Pulse C"() -> (w273:refnum<vi>)
  n382 = control-ref of="time to wait for solution change (min)"() -> (w428:refnum<vi>)
  n383 = control-ref of="time of Last V1 Change"() -> (w427:refnum<vi>)
  n384 = control-ref of="time of Last V2 Change"() -> (w426:refnum<vi>)
  n385 = control-ref of="time of Last V3 Change"() -> (w425:refnum<vi>)
  n386 = control-ref of="How Many Experimental Phases?"() -> (w451:refnum<vi>)
  n387 = Bundle(cluster="PhaseX Cluster", "Phase Experiment Option"=w362, "Paired Pulse"=w192, "Jump Train"=w191, "Voltage Ramp"=w190, "Voltage Step"=w189, "Solution Change"=w188, "Single Jump"=w187, "Single Manip Jump"=w186, "Gap Free"=w185, "Multi Manip Jump"=w184, "Voltage Pulse"=w183, "Current Pulse"=w58, "Current Ramp"=w57, "Gap Free Iclamp"=w56) -> (w356:T1)
  n388 = Bundle(cluster="PhaseX Cluster", "Phase Experiment Option"=w446, "Paired Pulse"=w282, "Jump Train"=w281, "Voltage Ramp"=w280, "Voltage Step"=w279, "Solution Change"=w278, "Single Jump"=w277, "Single Manip Jump"=w276, "Gap Free"=w275, "Multi Manip Jump"=w274, "Voltage Pulse"=w273, "Current Pulse"=w64, "Current Ramp"=w63, "Gap Free Iclamp"=w62) -> (w445:T1)
  n389 = control-ref of="Paired Pulse J"() -> (w173:refnum<vi>)
  n390 = control-ref of="Single Manip Jump J"() -> (w179:refnum<vi>)
  n391 = control-ref of="Voltage Ramp J"() -> (w175:refnum<vi>)
  n392 = control-ref of="Voltage Step J"() -> (w176:refnum<vi>)
  n393 = control-ref of="Solution Change J"() -> (w177:refnum<vi>)
  n394 = control-ref of="Single Jump J"() -> (w178:refnum<vi>)
  n395 = control-ref of="Jump Train J"() -> (w174:refnum<vi>)
  n396 = control-ref of="Gap Free J"() -> (w180:refnum<vi>)
  n397 = control-ref of="Multi Manip Jump J"() -> (w181:refnum<vi>)
  n398 = control-ref of="Voltage Pulse J"() -> (w182:refnum<vi>)
  n399 = control-ref of="Current Pulse J"() -> (w55:refnum<vi>)
  n400 = control-ref of="Current Ramp J"() -> (w54:refnum<vi>)
  n401 = control-ref of="Gap Free Iclamp J"() -> (w53:refnum<vi>)
  n402 = control-ref of="PhaseJ Experiment Option"() -> (w361:refnum<vi>)
  n403 = Bundle(cluster=T35 {"time of Last V1 Change"=refnum, "time of Last V2 Change"=refnum, "time of Last V3 Change"=refnum} ("valve Time Cluster"), "time of Last V1 Change"=w427, "time of Last V2 Change"=w426, "time of Last V3 Change"=w425) -> (w423:T35)
  n404 = control-ref of="PhaseD Experiment Option"() -> (w437:refnum<vi>)
  n405 = control-ref of="Current Pulse D"() -> (w61:refnum<vi>)
  n406 = control-ref of="Current Ramp D"() -> (w60:refnum<vi>)
  n407 = control-ref of="Gap Free Iclamp D"() -> (w59:refnum<vi>)
  n408 = control-ref of="Paired Pulse D"() -> (w262:refnum<vi>)
  n409 = control-ref of="Jump Train D"() -> (w261:refnum<vi>)
  n410 = control-ref of="Voltage Ramp D"() -> (w260:refnum<vi>)
  n411 = control-ref of="Voltage Step D"() -> (w259:refnum<vi>)
  n412 = control-ref of="Solution Change D"() -> (w258:refnum<vi>)
  n413 = control-ref of="Single Jump D"() -> (w257:refnum<vi>)
  n414 = control-ref of="Single Manip Jump D"() -> (w256:refnum<vi>)
  n415 = control-ref of="Gap Free D"() -> (w255:refnum<vi>)
  n416 = control-ref of="Multi Manip Jump D"() -> (w254:refnum<vi>)
  n417 = control-ref of="Voltage Pulse D"() -> (w253:refnum<vi>)
  n418 = Bundle(cluster="PhaseX Cluster", "Phase Experiment Option"=w361, "Paired Pulse"=w173, "Jump Train"=w174, "Voltage Ramp"=w175, "Voltage Step"=w176, "Solution Change"=w177, "Single Jump"=w178, "Single Manip Jump"=w179, "Gap Free"=w180, "Multi Manip Jump"=w181, "Voltage Pulse"=w182, "Current Pulse"=w55, "Current Ramp"=w54, "Gap Free Iclamp"=w53) -> (w355:T1)
  n419 = Bundle(cluster="PhaseX Cluster", "Phase Experiment Option"=w437, "Paired Pulse"=w262, "Jump Train"=w261, "Voltage Ramp"=w260, "Voltage Step"=w259, "Solution Change"=w258, "Single Jump"=w257, "Single Manip Jump"=w256, "Gap Free"=w255, "Multi Manip Jump"=w254, "Voltage Pulse"=w253, "Current Pulse"=w61, "Current Ramp"=w60, "Gap Free Iclamp"=w59) -> (w434:T1)
  n420 = control-ref of="Paired Pulse K"() -> (w172:refnum<vi>)
  n421 = control-ref of="Single Manip Jump K"() -> (w166:refnum<vi>)
  n422 = control-ref of="Voltage Ramp K"() -> (w170:refnum<vi>)
  n423 = control-ref of="Voltage Step K"() -> (w169:refnum<vi>)
  n424 = control-ref of="Solution Change K"() -> (w168:refnum<vi>)
  n425 = control-ref of="Single Jump K"() -> (w167:refnum<vi>)
  n426 = control-ref of="Jump Train K"() -> (w171:refnum<vi>)
  n427 = control-ref of="Gap Free K"() -> (w165:refnum<vi>)
  n428 = control-ref of="Current Pulse K"() -> (w46:refnum<vi>)
  n429 = control-ref of="Current Ramp K"() -> (w45:refnum<vi>)
  n430 = control-ref of="Gap Free Iclamp K"() -> (w44:refnum<vi>)
  n431 = control-ref of="Multi Manip Jump K"() -> (w164:refnum<vi>)
  n432 = control-ref of="Voltage Pulse K"() -> (w163:refnum<vi>)
  n433 = control-ref of="Phase A Done"() -> (w337:refnum<vi>)
  n434 = control-ref of="Phase B Done"() -> (w336:refnum<vi>)
  n435 = control-ref of="Phase C Done"() -> (w335:refnum<vi>)
  n436 = control-ref of="Phase D Done"() -> (w334:refnum<vi>)
  n437 = control-ref of="Phase E Done"() -> (w333:refnum<vi>)
  n438 = control-ref of="Phase F Done"() -> (w332:refnum<vi>)
  n439 = control-ref of="Phase G Done"() -> (w331:refnum<vi>)
  n440 = control-ref of="Phase H Done"() -> (w330:refnum<vi>)
  n441 = control-ref of="Phase I Done"() -> (w329:refnum<vi>)
  n442 = control-ref of="Phase J Done"() -> (w328:refnum<vi>)
  n443 = control-ref of="Phase K Done"() -> (w327:refnum<vi>)
  n444 = control-ref of="Phase L Done"() -> (w326:refnum<vi>)
  n445 = while {
    stop <- w519 stop-if-true
    n446 = local read "Puase for Loading"() -> (w518:bool)
    n447 = case shown="False" w518 {
      tunnel: [w523 FALSE] -> w519
      frame False {
        n448 = local read "auto WC run trigger"() -> (w520:bool)
        n449 = local write "auto WC run trigger"(w520) -> ()
        n450 = case shown="True" FALSE {
          frame False {
            n451 = Wait (ms)(milliseconds to wait=u32 1000) -> ()  [unwired: 1 out]
          }
          frame True {
            n452 = control-ref of="common cluster"() -> (w534:refnum<vi>)
            n453 = property class="Clust (strict)"(reference=w534) -> ("Value"=w533:T9)  [unwired: 1 in, 2 out]
            n454 = Unbundle By Name(w533) -> ("positioning+hunting common.transforms"=w537:refnum<vi>)
            n455 = property class="Clust (strict)"(reference=w537) -> (error out=w543:errorcluster, "Value"=w536:T36)  [unwired: 1 in, 1 out]
            n456 = Unbundle By Name(w536) -> ("manip 1"=w535:refnum<vi>)
            n457 = property class="Clust (strict)"(reference=w535, error in=w543) -> (error out=w544:errorcluster, "Value"=w541:T37)  [unwired: 1 out]
            n458 = Unbundle By Name(w541) -> ("actuator"=w542:T38)
            n459 = call "get_XYZ.vi"("Actuator cluster in"=w542, "error in"=w544) -> ("X pos (steps)"=w538:i32, "Y pos (steps)"=w539:i32, "Z pos (steps)"=w540:i32)  [unwired: 9 in, 2 out]
            n460 = Build Array(w538, w539, w540) -> (w530:i32[])
            n461 = Divide(x=w530, y=10) -> (x/y=w532:dbl[])
            n462 = To Long Integer(number=w532) -> (32bit integer=w529:i32[])
            "Current Manipulator Position [uM]" <- w529
            n463 = Wait (ms)(milliseconds to wait=u32 100) -> ()  [unwired: 1 out]
            n464 = stacked-sequence {
              tunnel: w533 -> [_ w563 w582 w601 w620 w639 w658 w677 w696 w715 w734 w753 w772 w791]
              tunnel: w529 -> [_ w546 w565 w587 w603 w622 w641 w660 w679 w698 w717 w736 w755 w774]
              frame #0 {
                n465 = local write "Current Position"("" ("Current Position")) -> ()
              }
              frame #1 {
                n466 = Unbundle By Name(w563) -> ("JumperPositions.jumperSafePos"=w562:refnum<vi>)
                n467 = property class="Arr (strict)"(reference=w562) -> ("Value"=w548:dbl[], "Caption.Text"=w551:string)  [unwired: 1 in, 2 out]
                n468 = Index Array(array=w546) -> (element #1=w560:i32, element #2=w558:i32, element #3=w557:i32)  [unwired: 3 in]
                n469 = Divide(x=w548, y=10) -> (x/y=w549:dbl[])
                n470 = To Long Integer(number=w549) -> (32bit integer=w547:i32[])
                n471 = Index Array(array=w547) -> (element #1=w561:i32, element #2=w559:i32, element #3=w556:i32)  [unwired: 3 in]
                n472 = Equal?(x=w561, y=w560) -> (x = y?=w555:bool)
                n473 = Equal?(x=w559, y=w558) -> (x = y?=w554:bool)
                n474 = Equal?(x=w556, y=w557) -> (x = y?=w553:bool)
                n475 = Compound Arithmetic op=AND(w555, w554, w553) -> (w552:bool)
                n476 = case shown="True" w552 {
                  tunnel: w551 -> [_ w564]
                  frame False {
                  }
                  frame True {
                    n477 = local write "Current Position"(w564) -> ()
                  }
                }
              }
              frame #2 {
                n478 = Unbundle By Name(w582) -> ("JumperPositions.ExpSafePos"=w581:refnum<vi>)
                n479 = property class="Arr (strict)"(reference=w581) -> ("Value"=w567:dbl[], "Caption.Text"=w570:string)  [unwired: 1 in, 2 out]
                n480 = Index Array(array=w565) -> (element #1=w579:i32, element #2=w577:i32, element #3=w576:i32)  [unwired: 3 in]
                n481 = Divide(x=w567, y=10) -> (x/y=w568:dbl[])
                n482 = To Long Integer(number=w568) -> (32bit integer=w566:i32[])
                n483 = Index Array(array=w566) -> (element #1=w580:i32, element #2=w578:i32, element #3=w575:i32)  [unwired: 3 in]
                n484 = Equal?(x=w580, y=w579) -> (x = y?=w574:bool)
                n485 = Equal?(x=w578, y=w577) -> (x = y?=w573:bool)
                n486 = Equal?(x=w575, y=w576) -> (x = y?=w572:bool)
                n487 = Compound Arithmetic op=AND(w574, w573, w572) -> (w571:bool)
                n488 = case shown="True" w571 {
                  tunnel: w570 -> [_ w583]
                  frame False {